vi "Login.vi"() -> ()   [LabVIEW 2020]
uses:
  System.Windows.Forms
  Global_Variable/Global.vi
  <userlib>/_MGI/Menu Building/MenuItemStatusChange/MGI_MenuItemStatusChange.lvclass
panel:
  in  "pwd":string
  in  "联机模式":enum16{"单机", "追溯"}(ring)
  in  "菜单":refnum<k24>(container)
  in  "登陆":bool
  in  "密   码":string
  in  "用户名":string
  out "数据库连接成功":bool
  # "滑移力复测及管柱总成装配台"
  # "数据库状态"
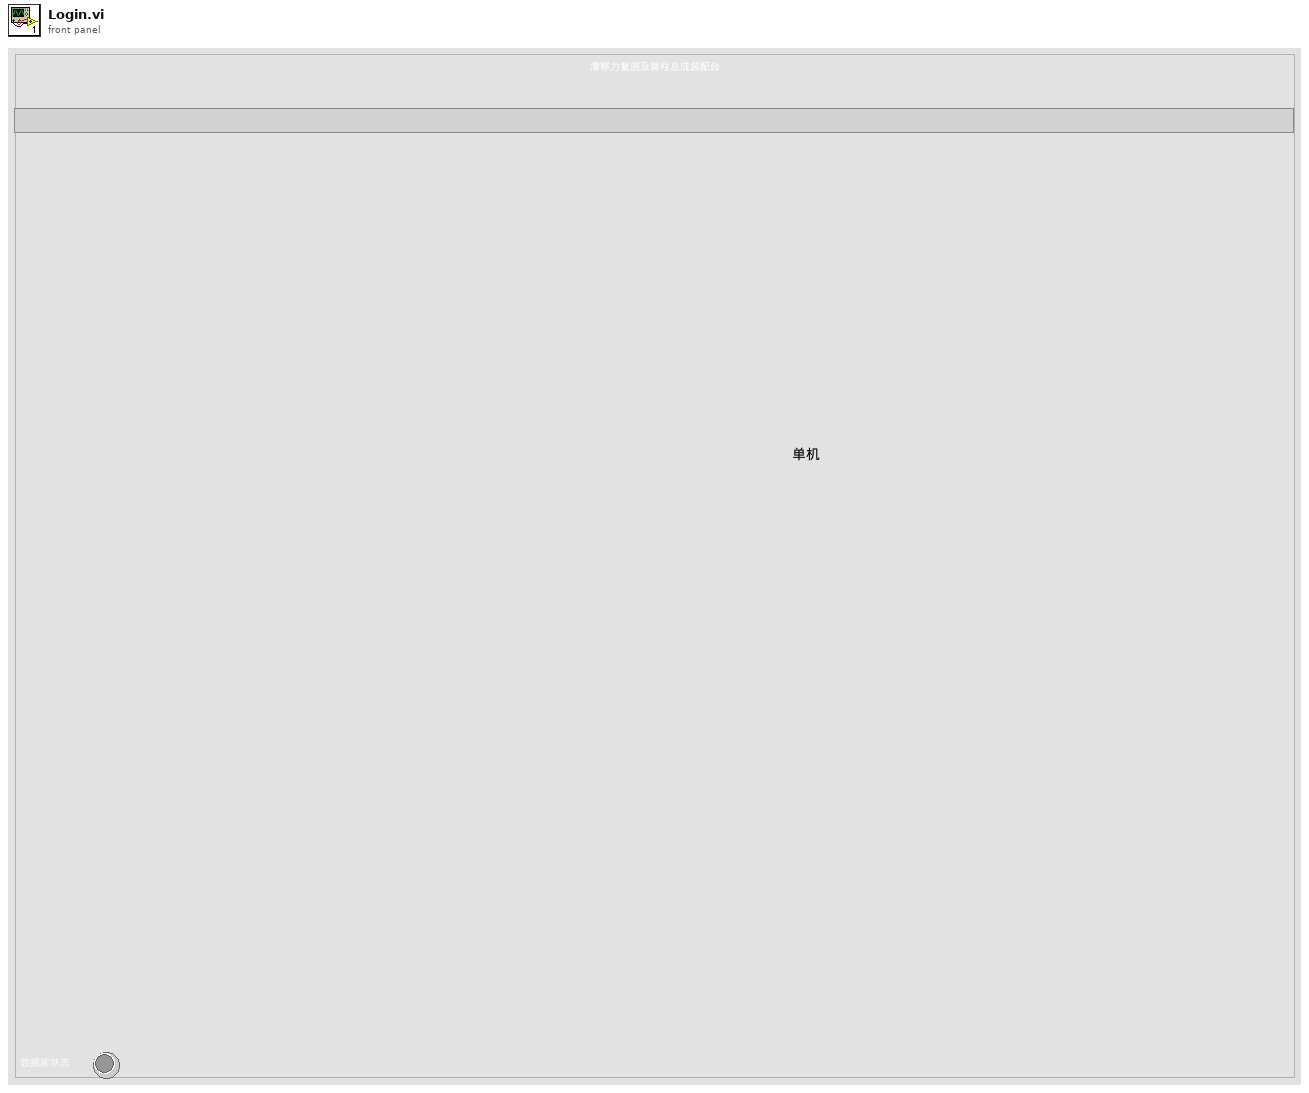
[diagram p1: front panel]
types:
  T1 = enum8{"Enabled", "Disabled", "Disabled and Grayed Out"}
  T2 = enum32{"Invalid", "Standard", "Closed", "Hidden", "Minimized", "Maximized"}
  T3 = cluster{"data[0]":string, "data[1]":string, "data[2]":string, "data[3]":string}
  T4 = typedef "eventvkey.ctl" = enum16{"ASCII", "Enter", "Return", "Shift", "Ctrl", "Alt", "Cmd", "Opt", "Caps", "NumLock", "Clear", "Break", "Up", "Down", "Left", "Right", "Insert", "Delete", "Home", "End", "PageUp", "PageDown", "Escape", "Help", "Pause", "ScrollLock", "F1", "F2", "F3", "F4", "F5", "F6", "F7", "F8", "F9", "F10", "F11", "F12", "F13", "F14", "F15", "F16", "F17", "F18", "F19", "F20", "F21", "F22", "F23", "F24", "Play", "VolumeUp", "VolumeDown", "Mute", "Two Byte Char"}
  T5 = cluster{"用户编号":string, "用户名":string, "用户密码(密文)":string, "用户权限":string}
  T6 = cluster{"操作员编号":string, "操作员姓名":string, "操作员权限":string, "联机模式":enum16{"单机", "追溯"}}
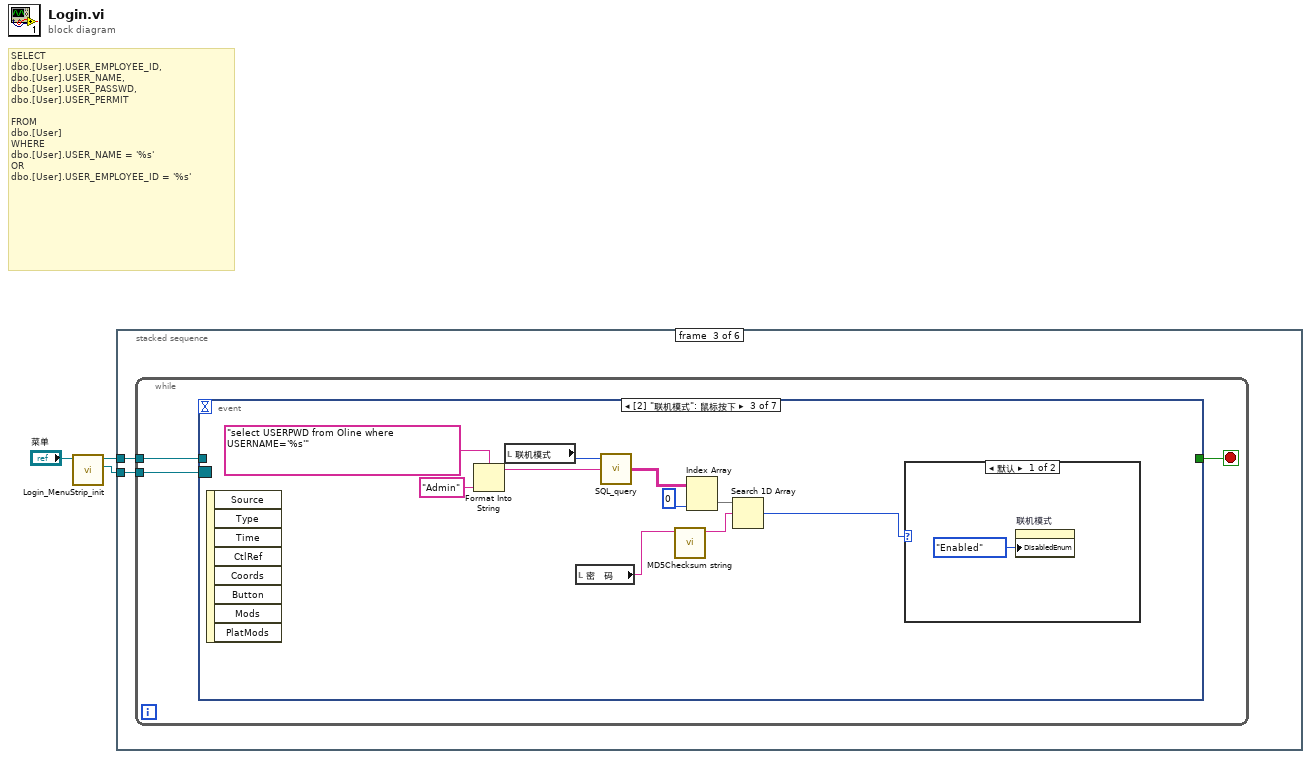
[diagram p0: block diagram]
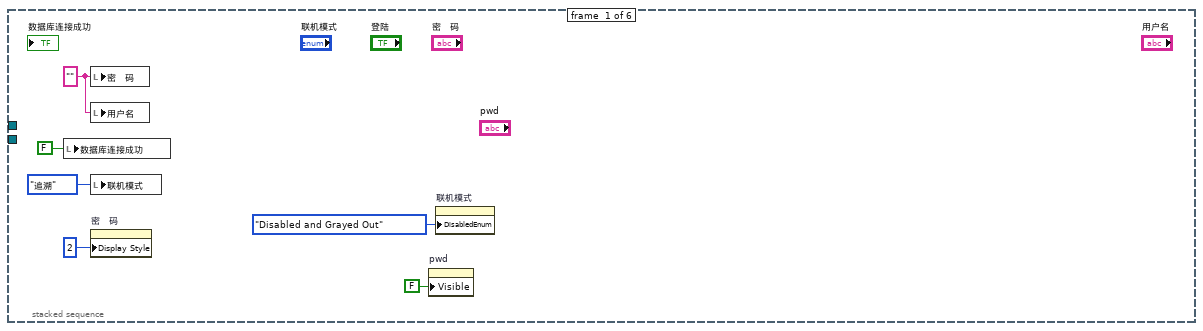
[diagram p2: hidden frame]
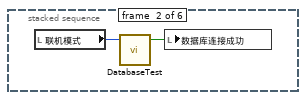
[diagram p3: hidden frame]
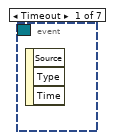
[diagram p4: hidden frame]
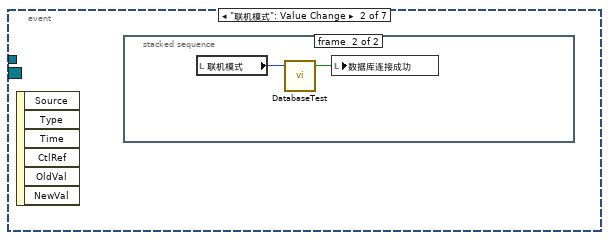
[diagram p5: hidden frame]
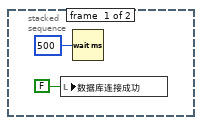
[diagram p6: hidden frame]
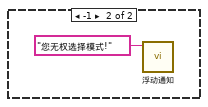
[diagram p7: hidden frame]
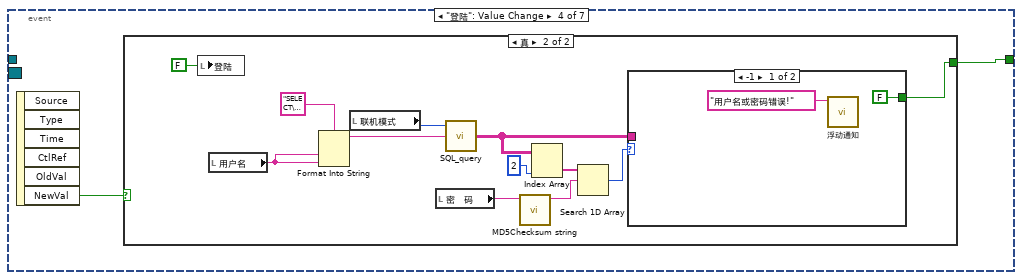
[diagram p8: hidden frame]
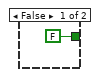
[diagram p9: hidden frame]
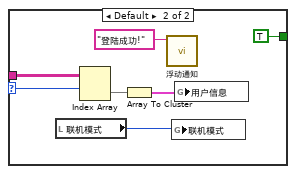
[diagram p10: hidden frame]
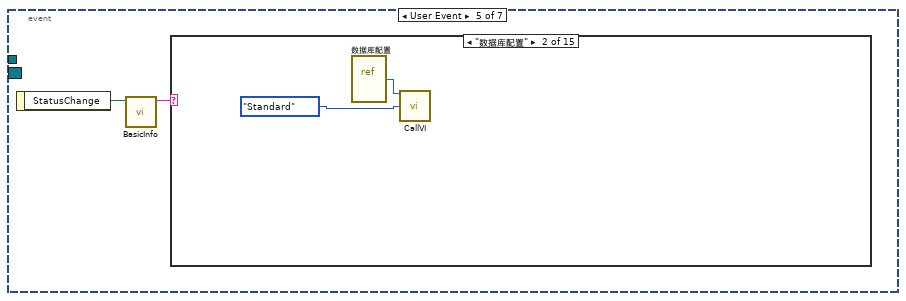
[diagram p11: hidden frame]
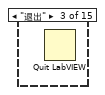
[diagram p13: hidden frame]
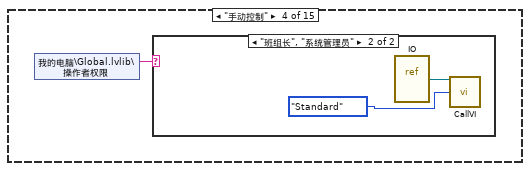
[diagram p14: hidden frame]
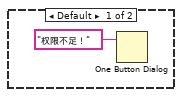
[diagram p15: hidden frame]
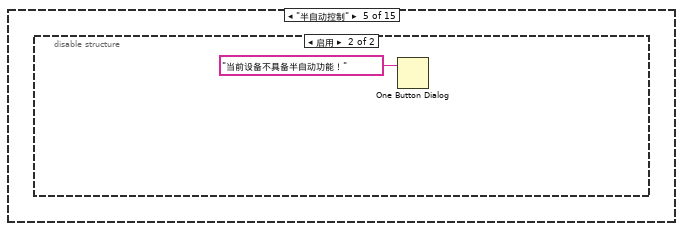
[diagram p16: hidden frame]
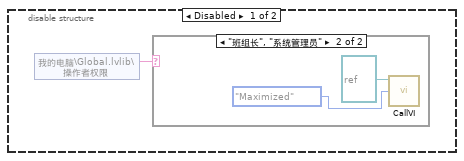
[diagram p17: hidden frame]
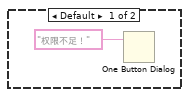
[diagram p18: hidden frame]
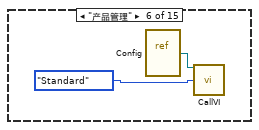
[diagram p19: hidden frame]
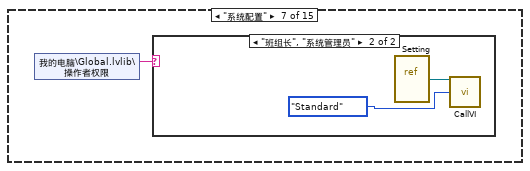
[diagram p20: hidden frame]
diagram:
  # "SELECT\ndbo.[User].USER_EMPLOYEE_ID,\ndbo.[User].USER_NAME,\ndbo.[User].USER_PASSWD,\ndbo.[User].USER_PERMIT\n\nFROM\ndbo.[User]\nWHERE\ndbo.[User].USER_NAME = '%s' \nOR\ndbo.[User].USER_EMPLOYEE_ID = '%s'"
  n1 = call "Login_MenuStrip_init.vi"("MenuStrip"="菜单") -> ("MenuStrip_Event"=w2:refnum<event-registration>, "Menu out"=w1:refnum<class "MGI_MenuStrip.lvclass">)  [unwired: 9 in]
  n2 = stacked-sequence {
    tunnel: w2 -> [_ _ w13 _ _ _]
    tunnel: w1 -> [_ _ w12 _ _ _]
    frame #0 {
      w8 = ""
      n3 = local write "数据库连接成功"(FALSE ("数据库连接成功")) -> ()
      n4 = local write "密   码"(w8) -> ()
      n5 = local write "用户名"(w8) -> ()
      n6 = local write "联机模式"(enum16{"单机", "追溯"}."追溯" ("联机模式")) -> ()
      n7 = property on="密   码" class="Str"("Display Style"=u32 2 ("显示样式")) -> ()  [unwired: 2 in, 2 out]
      n8 = property on="pwd" class="Str"("Visible"=FALSE ("可见")) -> ()  [unwired: 2 in, 2 out]
      n9 = property on="联机模式" class="Enum (严格)"("DisabledEnum"=T1."Disabled and Grayed Out" ("禁用")) -> ()  [unwired: 2 in, 2 out]
    }
    frame #1 {
      n10 = local read "联机模式"() -> (w10:enum16{"单机", "追溯"})
      n11 = call "DatabaseTest.vi"("联机模式"=w10) -> ("数据库连接成功"=w11:bool)  [unwired: 3 in, 1 out]
      n12 = local write "数据库连接成功"(w11) -> ()
    }
    frame #2 {
      n13 = while {
        tunnel: w13 -> [w15]
        tunnel: w12 -> [w14]
        stop <- w16 stop-if-true
        n14 = event shown="[2] \"联机模式\": 鼠标按下" {
          selector: w15 -> [_ _ _ _ _ _ _]
          dyn-events: _ -> [_ _ _ _ _ _ _]
          timeout: _ -> [_ _ _ _ _ _ _]
          tunnel: [_ _ _ w33 _ _ TRUE] -> w16
          tunnel: w14 -> [_ _ _ _ _ _ _]
          event Timeout {
            n15 = event-data() -> ()  [unwired: 1 in, 3 out]
          }
          event "联机模式": Value Change {
            n16 = event-data() -> ()  [unwired: 1 in, 6 out]
            n17 = stacked-sequence {
              frame #0 {
                n18 = local write "数据库连接成功"(FALSE ("数据库连接成功")) -> ()
                n19 = Wait (ms)(milliseconds to wait=u32 500 ("等待时间（毫秒）")) -> ()  [unwired: 1 out]
              }
              frame #1 {
                n20 = local read "联机模式"() -> (w19:enum16{"单机", "追溯"})
                n21 = call "DatabaseTest.vi"("联机模式"=w19) -> ("数据库连接成功"=w20:bool)  [unwired: 3 in, 1 out]
                n22 = local write "数据库连接成功"(w20) -> ()
              }
            }
          }
          event "联机模式": Mouse Down {
            n23 = event-data() -> ()  [unwired: 1 in, 8 out]
            n24 = Format Into String(format string="select USERPWD from Oline where USERNAME='%s'" ("格式字符串"), "Admin" ("输入 1")) -> (resulting string=w28:string)  [unwired: 2 in, 1 out]
            n25 = local read "联机模式"() -> (w26:enum16{"单机", "追溯"})
            n26 = local read "密   码"() -> (w21:string)
            n27 = call "SQL_query.vi"("SQL query"=w28, "联机模式"=w26) -> ("data"=w27:string[][])  [unwired: 2 in, 1 out]
            n28 = call <vilib>:"MD5Checksum string.vi"("Message String"=w21) -> ("MD5 message-digest"=w30:string)  [unwired: 10 in]
            n29 = Index Array(array=w27, index (col)=0 ("禁用的索引 (列)")) -> (element=w29:string[])  [unwired: 1 in]
            n30 = Search 1D Array(1D array=w29, element=w30) -> (index of element=w23:i32)  [unwired: 1 in]
            n31 = case shown="默认" w23 {
              frame Default {
                n32 = property on="联机模式" class="Enum (严格)"("DisabledEnum"=T1."Enabled" ("禁用")) -> ()  [unwired: 2 in, 2 out]
              }
              frame -1 {
                n33 = call "浮动通知.vi"("通知内容"="您无权选择模式!") -> ()  [unwired: 11 in]
              }
            }
          }
          event "登陆": Value Change {
            n34 = event-data() -> ("NewVal"=w34:bool)  [unwired: 1 in, 5 out]
            n35 = case shown="真" w34 {
              tunnel: [FALSE w38] -> w33
              frame False {
              }
              frame True {
                n36 = local write "登陆"(FALSE ("确定")) -> ()
                n37 = local read "用户名"() -> (w44:string)
                n38 = Format Into String(format string="SELECT\ndbo.[User].USER_EMPLOYEE_ID,\ndbo.[User].USER_NAME,\ndbo.[User].USER_PASSWD,\ndbo.[User].USER_PERMIT\n\nFROM\ndbo.[User]\nWHERE\ndbo.[User].USER_NAME = '%s' \nOR\ndbo.[User].USER_EMPLOYEE_ID = '%s'\n" ("格式字符串"), w44, w44) -> (resulting string=w41:string)  [unwired: 2 in, 1 out]
                n39 = local read "联机模式"() -> (w36:enum16{"单机", "追溯"})
                n40 = local read "密   码"() -> (w45:string)
                n41 = call "SQL_query.vi"("SQL query"=w41, "联机模式"=w36) -> ("data"=w39:string[][])  [unwired: 2 in, 1 out]
                n42 = call <vilib>:"MD5Checksum string.vi"("Message String"=w45) -> ("MD5 message-digest"=w46:string)  [unwired: 10 in]
                n43 = Index Array(array=w39, index (col)=2 ("禁用的索引 (列)")) -> (element=w43:string[])  [unwired: 1 in]
                n44 = Search 1D Array(1D array=w43, element=w46) -> (index of element=w40:i32)  [unwired: 1 in]
                n45 = case shown="-1" w40 {
                  selector: w40 -> [_ w55]
                  tunnel: w39 -> [_ w56]
                  tunnel: [FALSE TRUE] -> w38
                  frame -1 {
                    n46 = call "浮动通知.vi"("通知内容"="用户名或密码错误!") -> ()  [unwired: 11 in]
                  }
                  frame Default {
                    n47 = local read "联机模式"() -> (w51:enum16{"单机", "追溯"})
                    n48 = Index Array(array=w56, index (row)=w55) -> (element=w53:string[])  [unwired: 1 in]
                    n49 = Array To Cluster(array=w53) -> (cluster=w50:T3)
                    n50 = call "浮动通知.vi"("通知内容"="登陆成功!") -> ()  [unwired: 11 in]
                    n51 = global write "Global.vi" "联机模式"(w51) -> ()
                    n52 = global write "Global.vi" "用户信息"(w50) -> ()
                  }
                }
              }
            }
          }
          event User Event {
            n53 = event-data() -> ("StatusChange"=w58:refnum<class "MGI_MenuItemStatusChange.lvclass">)  [unwired: 1 in]
            n54 = call <userlib>:"BasicInfo.vi"("MGI_MenuItemStatusChange in"=w58) -> ("Tag"=w57:string)  [unwired: 7 in, 3 out]
            n55 = case shown="\"数据库配置\"" w57 {
              frame "假", Default {
              }
              frame "数据库配置" {
                n56 = vi-ref "数据库配置.vi"() -> (w60:refnum<vi>)
                n57 = call "CallVI.vi"("VI引用"=w60, "状态"=T2."Standard") -> ()  [unwired: 12 in, 2 out]
              }
              frame "退出" {
                n58 = Quit LabVIEW() -> ()  [unwired: 1 in]
              }
              frame "手动控制" {
                n59 = shared-variable "我的电脑\\Global.lvlib\\操作者权限"() -> (w61:string)  [unwired: 1 in, 1 out]
                n60 = case shown="\"班组长\", \"系统管理员\"" w61 {
                  frame Default {
                    n61 = One Button Dialog(message="权限不足！" ("消息")) -> ()  [unwired: 1 in, 1 out]
                  }
                  frame "班组长", "系统管理员" {
                    n62 = vi-ref "IO.vi"() -> (w64:refnum<vi>)
                    n63 = call "CallVI.vi"("VI引用"=w64, "状态"=T2."Standard") -> ()  [unwired: 12 in, 2 out]
                  }
                }
              }
              frame "半自动控制" {
                n64 = disable-structure shown="启用" {
                  frame Disabled {
                    n65 = shared-variable "我的电脑\\Global.lvlib\\操作者权限"() -> (w65:string)  [unwired: 1 in, 1 out]
                    n66 = case shown="\"班组长\", \"系统管理员\"" w65 {
                      frame Default {
                        n67 = One Button Dialog(message="权限不足！" ("消息")) -> ()  [unwired: 1 in, 1 out]
                      }
                      frame "班组长", "系统管理员" {
                        n68 = call "CallVI.vi"("VI引用"=refnum<vi> refnum, "状态"=T2."Maximized") -> ()  [unwired: 12 in, 2 out]
                      }
                    }
                  }
                  frame Enabled {
                    n69 = One Button Dialog(message="当前设备不具备半自动功能！" ("消息")) -> ()  [unwired: 1 in, 1 out]
                  }
                }
              }
              frame "产品管理" {
                n70 = vi-ref "Config.vi"() -> (w71:refnum<vi>)
                n71 = call "CallVI.vi"("VI引用"=w71, "状态"=T2."Standard") -> ()  [unwired: 12 in, 2 out]
              }
              frame "系统配置" {
                n72 = shared-variable "我的电脑\\Global.lvlib\\操作者权限"() -> (w72:string)  [unwired: 1 in, 1 out]
                n73 = case shown="\"班组长\", \"系统管理员\"" w72 {
                  frame Default {
                    n74 = One Button Dialog(message="权限不足！" ("消息")) -> ()  [unwired: 1 in, 1 out]
                  }
                  frame "班组长", "系统管理员" {
                    n75 = vi-ref "Setting.vi"() -> (w75:refnum<vi>)
                    n76 = call "CallVI.vi"("VI引用"=w75, "状态"=T2."Standard") -> ()  [unwired: 12 in, 2 out]
                  }
                }
              }
              frame "用户管理" {
                n77 = shared-variable "我的电脑\\Global.lvlib\\操作者权限"() -> (w76:string)  [unwired: 1 in, 1 out]
                n78 = case shown="\"系统管理员\"" w76 {
                  frame Default {
                    n79 = One Button Dialog(message="权限不足！" ("消息")) -> ()  [unwired: 1 in, 1 out]
                  }
                  frame "系统管理员" {
                    n80 = vi-ref "User_manager.vi"() -> (w79:refnum<vi>)
                    n81 = call "CallVI.vi"("VI引用"=w79, "状态"=T2."Standard") -> ()  [unwired: 12 in, 2 out]
                  }
                }
              }
              frame "编码规则" {
                n82 = shared-variable "我的电脑\\Global.lvlib\\操作者权限"() -> (w80:string)  [unwired: 1 in, 1 out]
                n83 = case shown="\"班组长\", \"工艺管理员\", \"系统管理员\"" w80 {
                  frame Default {
                    n84 = One Button Dialog(message="权限不足！" ("消息")) -> ()  [unwired: 1 in, 1 out]
                  }
                  frame "班组长", "工艺管理员", "系统管理员" {
                    n85 = vi-ref "编码规则设置.vi"() -> (w83:refnum<vi>)
                    n86 = call "CallVI.vi"("VI引用"=w83, "状态"=T2."Standard") -> ()  [unwired: 12 in, 2 out]
                  }
                }
              }
              frame "易损件管理" {
                n87 = vi-ref "易损件管理.vi"() -> (w85:refnum<vi>)
                n88 = call "CallVI.vi"("VI引用"=w85, "状态"=T2."Standard") -> ()  [unwired: 12 in, 2 out]
              }
              frame "物料批次管理" {
                n89 = vi-ref "批次管理.vi"() -> (w87:refnum<vi>)
                n90 = call "CallVI.vi"("VI引用"=w87, "状态"=T2."Standard") -> ()  [unwired: 12 in, 2 out]
              }
              frame "报表" {
                n91 = call "文件对话框"("start path"=path "D:/report", "prompt"="打开报表", "pattern (all files)"="*.doc;*.docx", "pattern label"="Word 文档") -> ("selected path"=w88:path, "error out"=w89:errorcluster)  [unwired: 8 in, 2 out]
                n92 = case shown="无错误" w89 {
                  selector: w89 -> [w95 w97]
                  tunnel: w88 -> [w96 _]
                  frame No Error {
                    w94 = 1 items=["Normal", "Maximize", "Minimize"] ("cpubbs_WindowState")
                    n93 = call "Open_Word.vi"("File Path"=w96, "cpubbs_WindowState"=w94, "错误输入（无错误）"=w95) -> ()  [unwired: 12 in, 1 out]
                  }
                  frame Error {
                    n94 = call <vilib>:"Clear Errors.vi"("error in (no error)"=w97) -> ()  [unwired: 5 in, 2 out]
                  }
                }
              }
              frame "报警信息" {
                n95 = vi-ref "报警信息.vi"() -> (w99:refnum<vi>)
                n96 = call "CallVI.vi"("VI引用"=w99, "状态"=T2."Standard") -> ()  [unwired: 12 in, 2 out]
              }
              frame "关于" {
                n97 = vi-ref "About.vi"() -> (w101:refnum<vi>)
                n98 = call "CallVI.vi"("VI引用"=w101, "状态"=T2."Standard") -> ()  [unwired: 12 in, 2 out]
              }
              frame "操作演示" {
                n99 = call <vilib>:"Application Directory.vi"() -> ("Application Directory"=w104:path)
                n100 = Build Path(base path=w104, name or relative path="操作演示" ("名称或相对路径")) -> (appended path=w103:path)
                n101 = call "自动播放ppt.vi"("路径"=w103) -> ()  [unwired: 10 in, 1 out]
              }
            }
          }
          event Key Down {
            n102 = event-data() -> ("VKey"=w105:T4)  [unwired: 1 in, 9 out]
            n103 = case shown="\"Return\"" w105 {
              frame "ASCII", Default {
              }
              frame "Return" {
                n104 = property on="登陆" class="Bool (严格)"("Val(Sgnl)"=TRUE ("值(信号)")) -> ()  [unwired: 2 in, 2 out]
              }
            }
          }
          event Panel Close {
            n105 = event-data() -> ()  [unwired: 1 in, 4 out]
            n106 = Quit LabVIEW() -> ()  [unwired: 1 in]
          }
        }
      }
    }
    frame #3 {
      n107 = global read "Global.vi" "用户信息"() -> (w111:T5)
      n108 = global read "用户信息.vi" "用户信息"() -> (w110:T6)
      n109 = Unbundle By Name(w111) -> ("用户编号"=w112:string, "用户权限"=w108:string)
      n110 = call "Get_Device_ID.vi"() -> ("Device_ID"=w114:string)  [unwired: 10 in, 1 out]
      n111 = Bundle By Name(cluster=w110, "操作员权限"=w108) -> (w109:T6)
      n112 = call "Get_USER_ID.vi"("USER_EMPLOYEE_ID"=w112) -> ("USER_ID"=w113:string)  [unwired: 9 in, 1 out]
      n113 = global write "追溯Global.vi" "DEVICE_ID"(w114) -> ()
      n114 = global write "用户信息.vi" "用户信息"(w109) -> ()
      n115 = global write "追溯Global.vi" "USER_ID"(w113) -> ()
    }
    frame #4 {
      n116 = vi-ref "Main.vi"() -> (w116:refnum<vi>)
      n117 = call "CallVI.vi"("VI引用"=w116, "状态"=T2."Maximized") -> ()  [unwired: 12 in, 2 out]
    }
    frame #5 {
      n118 = control-ref of="本VI"() -> (w117:refnum<vi>)
      n119 = invoke class="VI" method="FP.Close"(reference=w117) -> (reference out=w118:refnum<vi>, error out=w119:errorcluster)  [unwired: 2 in, 1 out]
      n120 = Close Reference(reference=w118, error in (no error)=w119) -> ()  [unwired: 1 out]
    }
  }
